vi "pharmaBot_v0.019.vi"() -> ()   [LabVIEW 2015] (continued)
  # "It saves the location when you push it -->"
  # "Set the Pipette Template"
  # "Click near the tip of the pipette in the @multiBot camera window then interface with the pop-up dialog to set the tip location and the pipette geometry.\n\nOnce complete, select the 'done' button below."
  # "Add Cells for Patching"
  # "Search around in the @multibot camera window and locate cells. Click on the center of desirable cells.\n\nOnce complete, select the 'done' button below."
  # "Calibration Complete"
  # "Stage"
  # "Manipulator"
  # "Select the Cell Index that you would like to add back into the \"unpatched cell indices\" array using the right and left arrow. To add the cell, click the Add Index to Unpatched Array Button. When finished, select done."
  # "CLEANING"
  # "EXPERIMENT SETTINGS"
  # "Voltage"
  # "NEURON DETECTION SETTINGS"
  # "Jumper"
  # "MACHINE VISION"
  # "DEBUGGING"
  # "MANIPULATOR 1"
  # "MANIPULATOR 2"
  # "CELL AUTOFOCUS"
  # "PIPETTE AUTOFOCUS"
  # "Position Set?"
  # "Jump Good?"
  # "HEK"
  # "SLICE"
  # "offset sets holding after membrane test..?"
  # "VERSION CONTROL\n\npharmaBot v0.009 - can't support dual patch but can control jumper\n\n9/9/17\nmultiBot v0.013 is compatible with multipatch_states_v0.013.\nColby's improved calibration routine is here. Adding pipette tracking verifier\n\n7/25/17\nmultiBot v0.011 is compatible with multipatch_states_v0.011: working on \ndual slice patching\n\n7-13-17\n- multiBot v0.010 is compatible with multipatch_states_v0.010. Latest stable version \nfor slice single patching and HEK cell dual patching\n\n7-6-17\nmultiBot v0.008 is compatible with multipatch_states_v0.008 AND v0.009\n- latest stable version - use for HEK and slices\n\n6/23/17\nmultiBot v0.007 is compatible with multipatch_states_v0.007\n- cell tracker working great\n- latest stable version for SINGLE-PATCH image tracking in slices\nmultiBot v0.006_reentrants is compatible with multipatch_states_wrapper_v0.001\nmultiBot v0.005 is compatible with multipatch_states_v0.005\nmultiBot v0.004 is compatible with multipatch_states_v0.004"
  # "TODO:\n\n- slow retractions for morphology\n- WC logic + recording software\n- simultaneous break-in\n- cell tracker for right pipette"
  # "@pharmaBot"
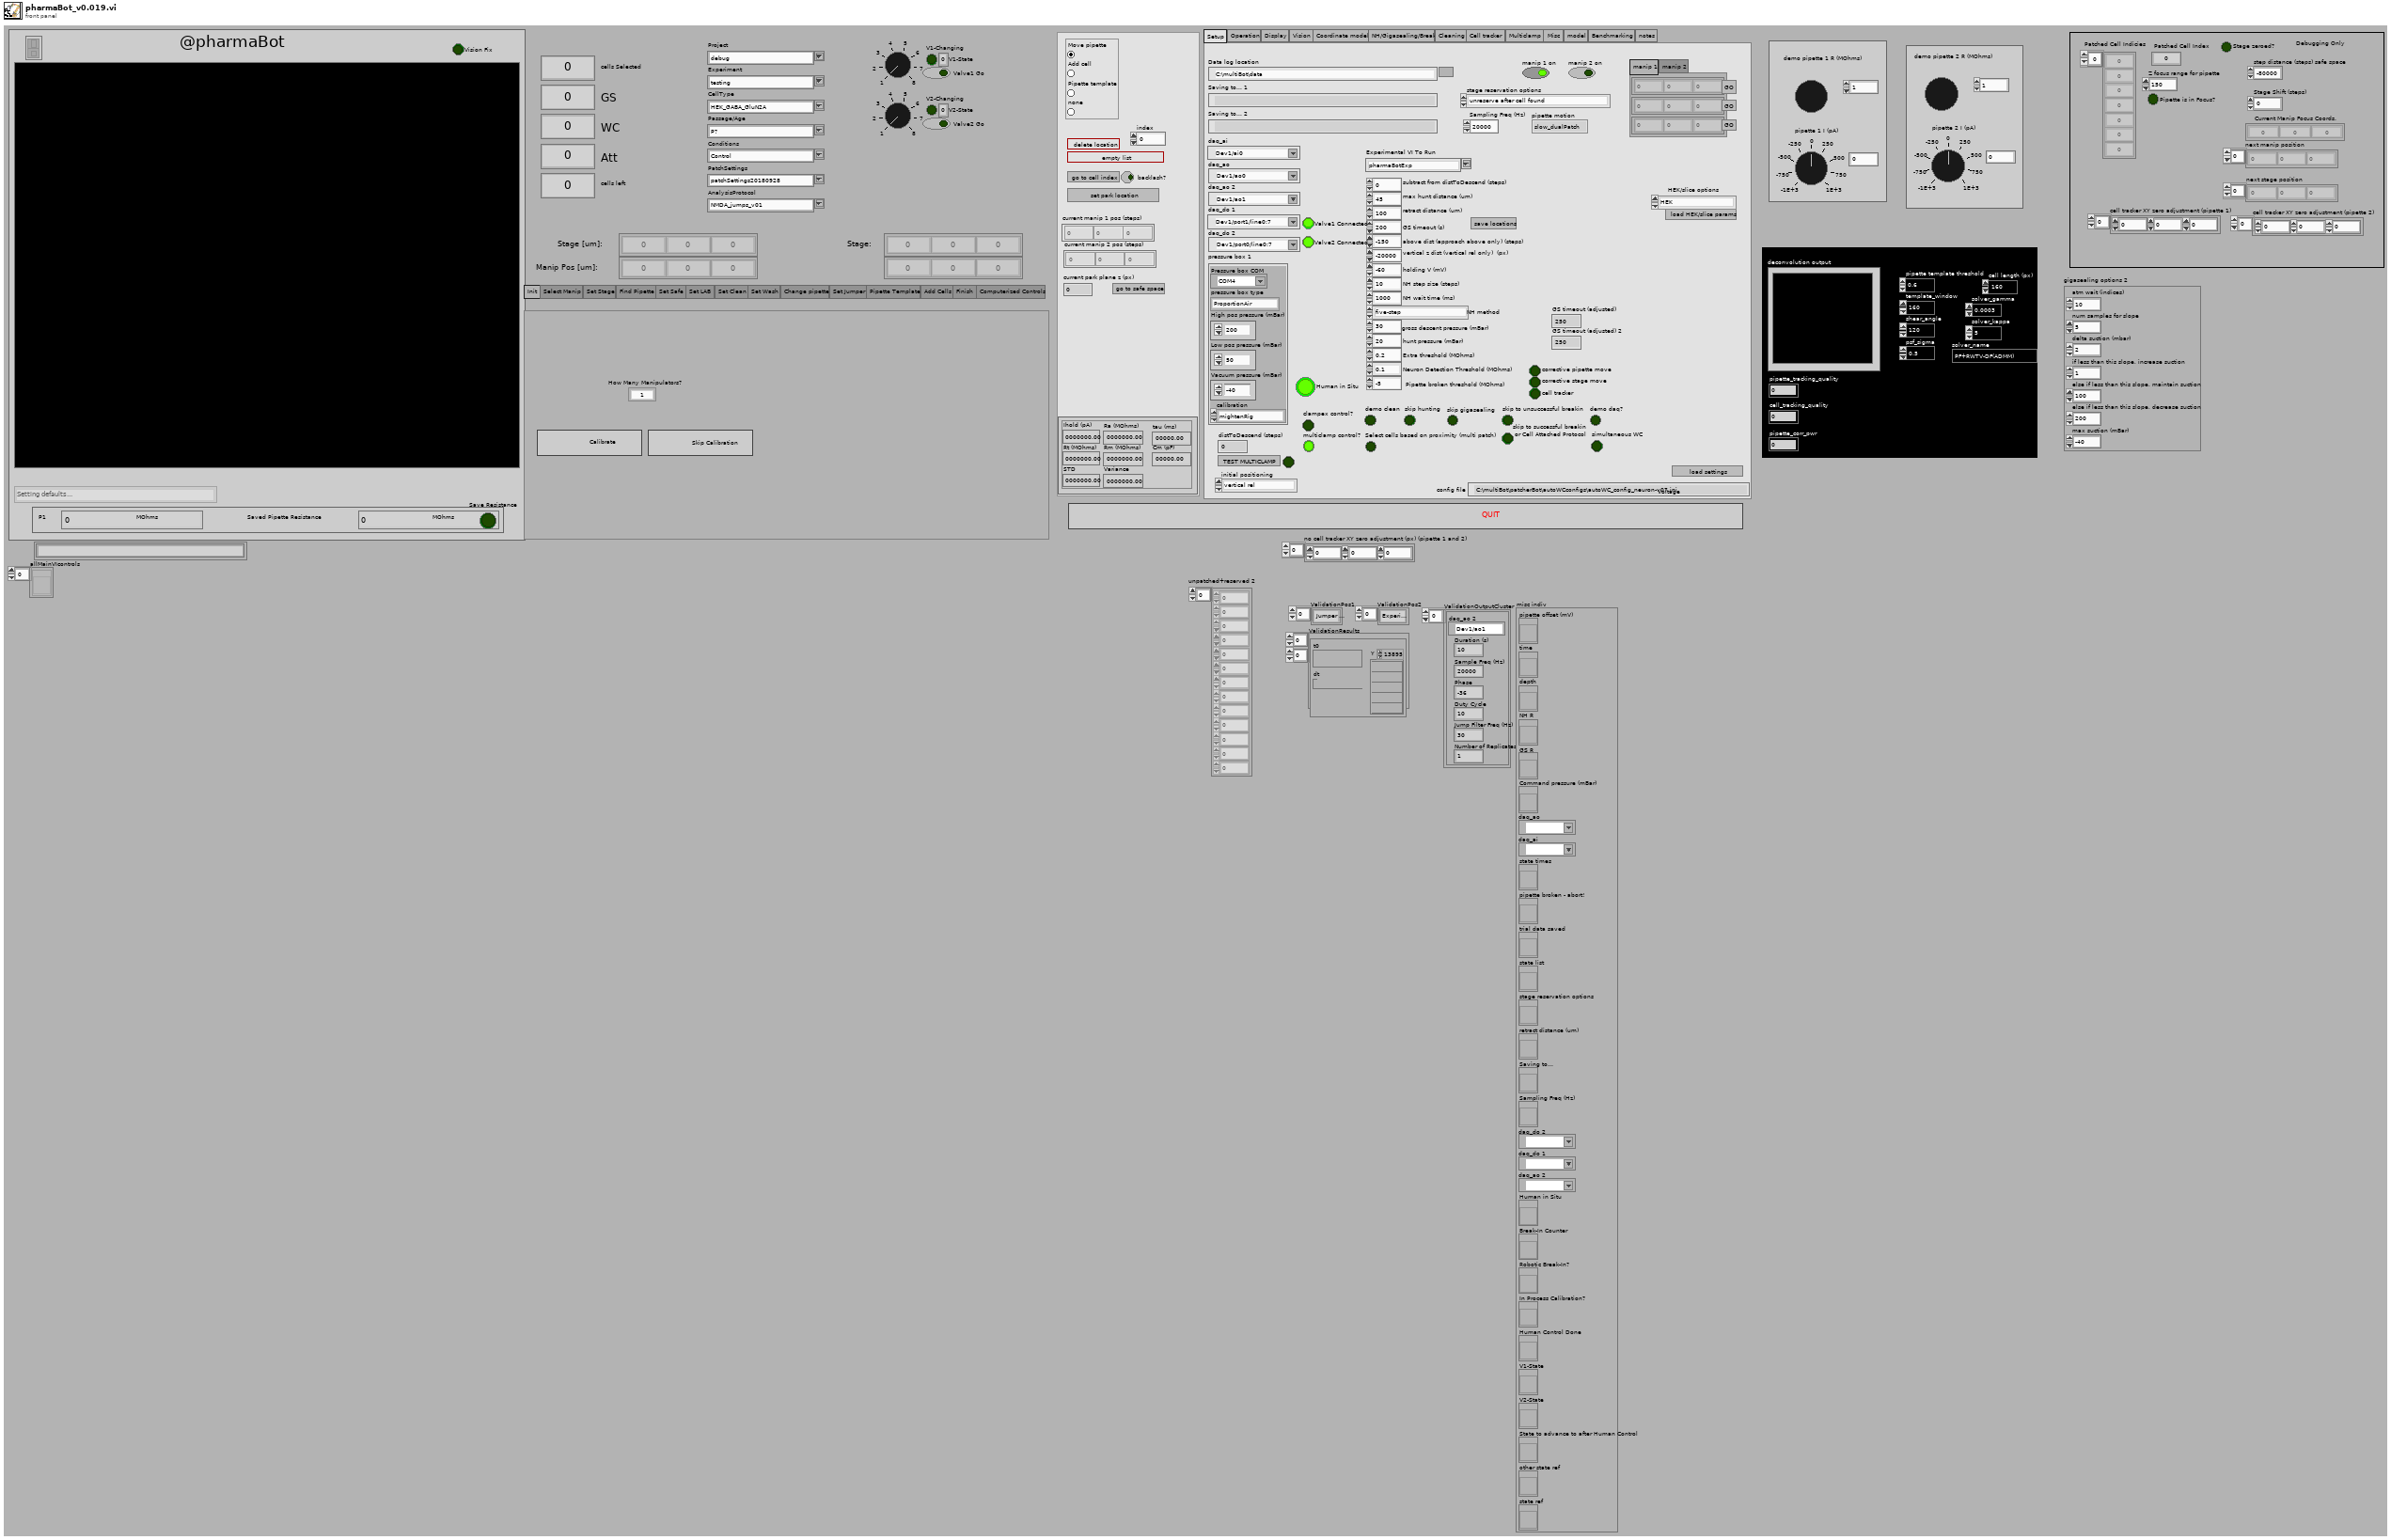
[diagram p1: front panel]
types:
  T1 = cluster{"pipette offset (mV)":refnum<vi>, "time":refnum<vi>, "depth":refnum<vi>, "NH R":refnum<vi>, "GS R":refnum<vi>, "Command pressure (mBar)":refnum<vi>, "daq_ao":tag, "daq_ai":tag, "state times":refnum<vi>, "pipette broken - abort!":refnum<vi>, "trial data saved":refnum<vi>, "state list":refnum<vi>, "stage reservation options":refnum<vi>, "retract distance (um)":refnum<vi>, "Saving to...":refnum<vi>, "Sampling Freq (Hz)":refnum<vi>, "daq_do 2":tag, "daq_do 1":tag, "daq_ao 2":tag, "Human in Situ":refnum<vi>, "Break-In Counter":refnum<vi>, "Robotic Break-In?":refnum<vi>, "In Process Calibration?":refnum<vi>, "Human Control Done":refnum<vi>, "V1-State":refnum<vi>, "V2-State":refnum<vi>, "State to advance to after Human Control":refnum<vi>, "other state ref":refnum<vi>, "state ref":refnum<vi>}
  T2 = cluster{"daq_ao 2":tag, "Duration (s)":dbl, "Sample Freq (Hz)":dbl, "Phase":dbl, "Duty Cycle":dbl, "Jump Filter Freq (Hz)":dbl, "Number of Replicates":i16}[]
  T3 = enum16{"Jumper Safe Position", "Experiment Safe Position", "Jumper Position A", "Jumper Position B", "Jumper Position C", "Jumper Position o-A", "Jumper Position A-o", "Jumper Position A-B", "Jumper Position B-A", "Jumper Position B-C", "Jumper Position C-B", "Jumper Position C-o", "Jumper Position o-C"}[]
  T4 = cluster{"atm wait (indices)":i32, "num samples for slope":i32, "delta suction (mbar)":dbl, "if less than this slope, increase suction":dbl, "else if less than this slope, maintain suction":dbl, "else if less than this slope, decrease suction ":dbl, "max suction (mBar)":dbl}
  T5 = typedef "cell_stats-v02.ctl" = cluster{"Ihold (pA)":dbl, "Rm (MOhms)":dbl, "Ra (MOhms)":dbl, "Cm (pF)":dbl, "tau (ms)":dbl, "Rt (MOhms)":dbl, "Variance":dbl, "STD":dbl}
  T6 = enum32{"Move pipette", "Add cell", "Pipette template", "none"}
  T7 = enum32{"Init", "Select Manip", "Set Stage", "Find Pipette", "Set Safe", "Set LAB", "Set Clean", "Set Wash", "Reset 0s", "Change pipette", "Set Jumper", "Pipette Template", "Add Cells", "Finish", "Computerized Controls", "Load Old Cells"}
  T8 = enum16{"manipulator 1", "manipulator 2", "manipulator 3", "manipulator 4"}
  T9 = enum16{"Jumper Safe Position", "Experiment Safe Position", "Jumper Position A", "Jumper Position B", "Jumper Position C", "Jumper Position o-A", "Jumper Position A-o", "Jumper Position A-B", "Jumper Position B-A", "Jumper Position B-C", "Jumper Position C-B", "Jumper Position C-o", "Jumper Position o-C"}
  T10 = typedef "IMAQ Image.ctl" = refnum<image>
  T11 = typedef "user_message_v6.ctl" = enum16{"Initializing...", "Setting defaults...", "Click OK to start patcherBot!", "Starting new attempt...", "Pipette repositioning...", "Initializing cell tracker...", "Gross approach...", "Human Positioning...", "In Process Calibration", "Detecting cell...", "Cell detected...", "Gigaseal Established...", "Breaking in...", "Successful breakin!", "Unsuccessful breakin!", "Whole-cell recording", "Saving autopatching parameters...", "Quitting VI", "Waiting for idle stage...", "Cleaning...", "Retracting pipette...", "DEBUG STATE", "Waiting to break in...", "Waiting for WC", "reclean", "Done with Current Set of Cells"}
  T12 = enum32{"Setup", "Operation", "Display", "Vision", "Coordinate model", "NH/Gigasealing/Break", "Cleaning", "Cell tracker", "Multiclamp", "Misc", "model", "Benchmarking", "notes"}
  T13 = typedef "Control 7b.ctl" = i32
  T14 = typedef "pressure_box_control.ctl" = cluster{"Pressure box COM":refnum<visa-resource-name>, "pressure box type":T15, "High pos pressure (mBar)":dbl, "Low pos pressure (mBar)":dbl, "Vacuum pressure (mBar)":dbl, "calibration":enum16{"PA_vacPump", "PA_venturi", "Neuromatics", "ilyaRig", "mightenRig"}}
  T15 = typedef "pressure_box_type.ctl" = enum16{"Neuromatics", "ProportionAir", "Demo box", "N-ProportionAir"}
  T16 = typedef "approach_type.ctl" = enum16{"right to cell", "vertical abs", "approach", "vertical rel", "approach above"}
  T17 = enum16{"unreserve after gross approach", "unreserve after cell found"}
  T18 = typedef "NH_method.ctl" = enum16{"five-step", "three-stepANDfixedCutOff", "three-step"}
  T19 = typedef "scope_motion.ctl" = enum16{"superSlow", "fast", "slow", "find slice speed", "slow_dualPatch"}
  T20 = typedef "notSureControl-v01.ctl" = bool
  T21 = cluster{"Starting Value":sgl, "Incremental Value":sgl, "Histogram":u32[]}
  T22 = typedef "cam_type-v02.ctl" = enum16{"HamamatsuORCA05G", "Qcam", "optiMOS"}
  T23 = cluster{"width x":dbl, "height y":dbl, "x offset":dbl, "y offset":dbl}
  T24 = enum32{"stage", "manip 1", "manip 2", "manip 3", "manip 4"}
  T25 = typedef "transform_properties_actuators.ctl" = cluster{"theta (deg)":dbl, "X sc factor (px/step)":dbl, "Y sc factor (px/step)":dbl, "zero loc (x,y,z)":dbl[], "flip y?":bool, "flip x?":bool, "gamma (deg)":dbl, "flip z?":bool, "Z sc factor (px/step)":dbl, "actuator":T26, "safe space (steps)":i32[]}
  T26 = typedef "actuator_cluster.ctl" = cluster{"Actuator COM":refnum<visa-resource-name>, "Actuator type":T27}
  T27 = typedef "actuator_type.ctl" = enum16{"Scientifica", "Sutter", "Demo", "Off"}
  T28 = typedef "ROI Descriptor" = cluster{"Global Rectangle":i32[], "Contours":cluster{"ID":enum32{"External", "Internal"}, "Type":u32, "Coordinates":i32[]}[]}
  T29 = typedef "memtest_def.ctl" = cluster{"Samples to Read":i32, "Rate (Hz)":dbl, "Amplitude (mV/pA)":dbl, "Offset (mV/pA)":dbl, "Frequency (Hz)":dbl, "duty cycle (%)":dbl, "phase":dbl}
  T30 = cluster{u32, string, i32, u32, u32, u32, "arg1":i32}
  T31 = enum16{"manipulator 1", "manipulator 2", "manipulator 3", "manipulator 4"}[]
  T32 = typedef "dual_patch_controls.ctl" = cluster{"sampling rate (Hz)":dbl, "total duration (s)":dbl, "stim amplitude (pA)":dbl, "time between stims (s)":dbl, "delta t (s)":dbl, "pulse width (s)":dbl, "# repetitions":dbl, "number of pulses":i32, "before stim (s)":dbl}
  T33 = cluster{"cells (image px locations)":dbl[], "cells (image px locations)":dbl[]}[]
  T34 = typedef "multipatch_individual_controls_v5.ctl" = cluster{"state UI indiv":cluster{"clampex control?":refnum<vi>, "demo clean":refnum<vi>, "skip hunting":refnum<vi>, "skip gigasealing":refnum<vi>, "multiclamp control?":refnum<vi>, "corrective pipette move":refnum<vi>, "corrective stage move":refnum<vi>, "cell tracker":refnum<vi>, "demo daq?":refnum<vi>, "skip to unsuccessful breakin":refnum<vi>, "skip to successful breakin":refnum<vi>, "successful breakin":refnum<vi>}, "positioning + hunting indiv":cluster{"NH step size (steps)":refnum<vi>, "hunt pressure (mBar)":refnum<vi>, "distToDescend (steps)":refnum<vi>, "approach above cell (steps)":refnum<vi>, "initial positioning":refnum<vi>, "d(above cell) (steps)":refnum<vi>, "neuron found":refnum<vi>, "NEURON HUNTING MONITOR":refnum<vi>, "Memtest inputs":refnum<vi>, "max hunt distance (um)":refnum<vi>, "Neuron Detection Threshold (MOhms)":refnum<vi>, "Pipette broken threshold (MOhms)":refnum<vi>, "gross descent pressure (mBar)":refnum<vi>, "Extra threshold (MOhms)":refnum<vi>, "current cell":refnum<vi>, "vertical z dist (vertical rel only)  (px)":refnum<vi>}, "gigaseal indiv":cluster{"GS timeout (s)":refnum<vi>, "GS timeout (adjusted)":refnum<vi>, "vhold applied?":refnum<vi>, "pipette resistance":refnum<vi>, "Iholding":refnum<vi>, "start GS time":refnum<vi>, "GIGASEALING MONITOR":refnum<vi>, "current Vholding (mV)":refnum<vi>, "GS extended":refnum<vi>, "holding V (mV)":refnum<vi>, "gigasealing options":refnum<vi>, "Cm":refnum<vi>, "Ra ":refnum<vi>}, "cleaning indiv":cluster{"pre-clean":refnum<vi>, "loc above baths":refnum<vi>, "wash bath loc":refnum<vi>, "cleaning bath loc":refnum<vi>, "cleaning status":refnum<vi>, "avg peak height":refnum<vi>, "clean bath detected":refnum<vi>, "wash bath detected":refnum<vi>}, "cell tracker indiv":cluster{"screen tip location (px)":refnum<vi>, "cell found":refnum<vi>, "tip found":refnum<vi>, "cell tracking box (px)":refnum<vi>}, "misc indiv":cluster{"pipette offset (mV)":refnum<vi>, "time":refnum<vi>, "depth":refnum<vi>, "NH R":refnum<vi>, "GS R":refnum<vi>, "Command pressure (mBar)":refnum<vi>, "daq_ao":tag, "daq_ai":tag, "state times":refnum<vi>, "pipette broken - abort!":refnum<vi>, "trial data saved":refnum<vi>, "state list":refnum<vi>, "stage reservation options":refnum<vi>, "retract distance (um)":refnum<vi>, "Saving to...":refnum<vi>, "Sampling Freq (Hz)":refnum<vi>, "daq_do 2":tag, "daq_do 1":tag, "daq_ao 2":tag, "Human in Situ":refnum<vi>, "Break-In Counter":refnum<vi>, "Robotic Break-In?":refnum<vi>, "In Process Calibration?":refnum<vi>, "Human Control Done":refnum<vi>, "V1-State":refnum<vi>, "V2-State":refnum<vi>, "State to advance to after Human Control":refnum<vi>, "other state ref":refnum<vi>, "state ref":refnum<vi>}, "breakin indiv":cluster{"breakin counter":refnum<vi>, "MAX Break In Pressure (mbar)":refnum<vi>}, "vision indiv":cluster{"manip position":refnum<vi>, "cell tracker XY zero adjustment (px)":refnum<vi>, "no cell tracker XY zero adjustment (px)":refnum<vi>}}
  T35 = cluster{"current stage pos (steps)":refnum<vi>, "current manip 1 pos (steps)":refnum<vi>, "current manip 2 pos (steps)":refnum<vi>, "current manip 3 pos (steps)":refnum<vi>, "current manip 4 pos (steps)":refnum<vi>}
  T36 = typedef "transform_cluster_actuator.ctl" = cluster{"s":refnum<vi>, "manip 1":refnum<vi>, "manip 2":refnum<vi>, "manip 3":refnum<vi>, "manip 4":refnum<vi>}
  T37 = typedef "multipatch_common_controls_v4.ctl" = cluster{"cell tracker common":cluster{"solver_beta":refnum<vi>, "solver_kappa":refnum<vi>, "shear_angle":refnum<vi>, "solver_gamma":refnum<vi>, "template_window":refnum<vi>, "debug_mode":refnum<vi>, "psf_sigma":refnum<vi>, "solver_name":refnum<vi>, "centroid_px":refnum<vi>, "pipette_px":refnum<vi>, "pipette_tracking_quality":refnum<vi>, "cell_tracking_quality":refnum<vi>, "pipette template threshold":refnum<vi>, "cell centroid array":refnum<vi>, "pipette centroid array":refnum<vi>, "cell length (px)":refnum<vi>}, "vision common":cluster{"init tracker success":refnum<vi>, "run tracker success":refnum<vi>, "tracking":refnum<vi>, "exit tracker success":refnum<vi>, "init error out":refnum<vi>, "current pipette locations (px)":refnum<vi>, "cell image size (px)":refnum<vi>, "pipette match score":refnum<vi>, "cell match score":refnum<vi>}, "misc common":cluster{"initialized":refnum<vi>, "Data log location":refnum<vi>, "Multiclamp Handle":refnum<vi>, "mclamp cluster":refnum<vi>, "User OK":refnum<vi>, "stage idle?":refnum<vi>, "stop":refnum<vi>, "pipette motion":refnum<vi>, "stop memtest":refnum<vi>, "dual patch cluster":refnum<vi>, "simultaneous WC":refnum<vi>, "Select cells based on proximity (multi patch)":refnum<vi>, "dual WC keep going":refnum<vi>, "HEK/slice options":refnum<vi>, "Terminate Experiment":refnum<vi>, "Validate":refnum<vi>}, "positioning+hunting common":cluster{"current cell locations (px)":refnum<vi>, "cells (image px)":refnum<vi>, "current park plane z (px)":refnum<vi>, "gross descent pressure (mBar)":refnum<vi>, "positions":refnum<vi>, "transforms":refnum<vi>, "pressure box":refnum<vi>, "current pipette locations (px)":refnum<vi>, "unpatched cell indices":refnum<vi>, "NH method":refnum<vi>, "NH wait time (ms)":refnum<vi>}, "ExperimentDescriptors":cluster{"Project":refnum<vi>, "AnalysisProtocol":refnum<vi>, "PatchSettings":refnum<vi>, "Passage/Age":refnum<vi>, "CellType":refnum<vi>, "Experiment":refnum<vi>, "Conditions":refnum<vi>, "ExperimentVIToRun":refnum<vi>}, "JumperPositions":cluster{"JumperPos o-C":refnum<vi>, "JumperPos C-o":refnum<vi>, "JumperPos C-B":refnum<vi>, "JumperPos B-C":refnum<vi>, "JumperPos B-A":refnum<vi>, "JumperPos A-B":refnum<vi>, "JumperPos A-o":refnum<vi>, "JumperPos o-A":refnum<vi>, "JumperPos C":refnum<vi>, "JumperPos B":refnum<vi>, "JumperPos A":refnum<vi>, "ExpSafePos":refnum<vi>, "jumperSafePos":refnum<vi>}, "PreviousValidationResults":cluster{"ValidationResults":refnum<vi>, "ValidationPos1":refnum<vi>, "ValidationPos2":refnum<vi>, "ValidationOutputCluster":refnum<vi>}}
  T38 = typedef "cam_info.ctl" = cluster{"camera type":T22, "cam handle":u32, "data handle":u32, "cam size":i32[]}
  T39 = cluster{"initialized":refnum<vi>, "Data log location":refnum<vi>, "Multiclamp Handle":refnum<vi>, "mclamp cluster":refnum<vi>, "User OK":refnum<vi>, "stage idle?":refnum<vi>, "stop":refnum<vi>, "pipette motion":refnum<vi>, "stop memtest":refnum<vi>, "dual patch cluster":refnum<vi>, "simultaneous WC":refnum<vi>, "Select cells based on proximity (multi patch)":refnum<vi>, "dual WC keep going":refnum<vi>, "HEK/slice options":refnum<vi>, "Terminate Experiment":refnum<vi>, "Validate":refnum<vi>}
  T40 = cluster{"init tracker success":refnum<vi>, "run tracker success":refnum<vi>, "tracking":refnum<vi>, "exit tracker success":refnum<vi>, "init error out":refnum<vi>, "current pipette locations (px)":refnum<vi>, "cell image size (px)":refnum<vi>, "pipette match score":refnum<vi>, "cell match score":refnum<vi>}
  T41 = cluster{"solver_beta":refnum<vi>, "solver_kappa":refnum<vi>, "shear_angle":refnum<vi>, "solver_gamma":refnum<vi>, "template_window":refnum<vi>, "debug_mode":refnum<vi>, "psf_sigma":refnum<vi>, "solver_name":refnum<vi>, "centroid_px":refnum<vi>, "pipette_px":refnum<vi>, "pipette_tracking_quality":refnum<vi>, "cell_tracking_quality":refnum<vi>, "pipette template threshold":refnum<vi>, "cell centroid array":refnum<vi>, "pipette centroid array":refnum<vi>, "cell length (px)":refnum<vi>}
  T42 = cluster{"Project":refnum<vi>, "AnalysisProtocol":refnum<vi>, "PatchSettings":refnum<vi>, "Passage/Age":refnum<vi>, "CellType":refnum<vi>, "Experiment":refnum<vi>, "Conditions":refnum<vi>, "ExperimentVIToRun":refnum<vi>}
  T43 = cluster{"current cell locations (px)":refnum<vi>, "cells (image px)":refnum<vi>, "current park plane z (px)":refnum<vi>, "gross descent pressure (mBar)":refnum<vi>, "positions":refnum<vi>, "transforms":refnum<vi>, "pressure box":refnum<vi>, "current pipette locations (px)":refnum<vi>, "unpatched cell indices":refnum<vi>, "NH method":refnum<vi>, "NH wait time (ms)":refnum<vi>}
  T44 = cluster{"GS timeout (s)":refnum<vi>, "GS timeout (adjusted)":refnum<vi>, "vhold applied?":refnum<vi>, "pipette resistance":refnum<vi>, "Iholding":refnum<vi>, "start GS time":refnum<vi>, "GIGASEALING MONITOR":refnum<vi>, "current Vholding (mV)":refnum<vi>, "GS extended":refnum<vi>, "holding V (mV)":refnum<vi>, "gigasealing options":refnum<vi>, "Cm 1":refnum<vi>, "Ra 1":refnum<vi>}
  T45 = cluster{"JumperPos o-C":refnum<vi>, "JumperPos C-o":refnum<vi>, "JumperPos C-B":refnum<vi>, "JumperPos B-C":refnum<vi>, "JumperPos B-A":refnum<vi>, "JumperPos A-B":refnum<vi>, "JumperPos A-o":refnum<vi>, "JumperPos o-A":refnum<vi>, "JumperPos C":refnum<vi>, "JumperPos B":refnum<vi>, "JumperPos A":refnum<vi>, "ExpSafePos":refnum<vi>, "jumperSafePos":refnum<vi>}
  T46 = cluster{"ValidationResults":refnum<vi>, "ValidationPos1":refnum<vi>, "ValidationPos2":refnum<vi>, "ValidationOutputCluster":refnum<vi>}
  T47 = typedef "Image Type" = u32
  T48 = cluster{"clampex control?":refnum<vi>, "demo clean":refnum<vi>, "skip hunting":refnum<vi>, "skip gigasealing":refnum<vi>, "multiclamp control?":refnum<vi>, "corrective pipette move":refnum<vi>, "corrective stage move":refnum<vi>, "cell tracker":refnum<vi>, "demo daq?":refnum<vi>, "skip to unsuccessful breakin":refnum<vi>, "skip to successful breakin":refnum<vi>, "successful breakin":refnum<vi>}
  T49 = cluster{"NH step size (steps)":refnum<vi>, "hunt pressure (mBar)":refnum<vi>, "distToDescend (steps)":refnum<vi>, "approach above cell (steps)":refnum<vi>, "initial positioning":refnum<vi>, "d(above cell) (steps)":refnum<vi>, "neuron found":refnum<vi>, "NEURON HUNTING MONITOR":refnum<vi>, "Memtest inputs":refnum<vi>, "max hunt distance (um)":refnum<vi>, "Neuron Detection Threshold (MOhms)":refnum<vi>, "Pipette broken threshold (MOhms)":refnum<vi>, "gross descent pressure (mBar)":refnum<vi>, "Extra threshold (MOhms)":refnum<vi>, "current cell":refnum<vi>, "vertical z dist (vertical rel only)  (px)":refnum<vi>}
  T50 = cluster{"pre-clean":refnum<vi>, "loc above baths":refnum<vi>, "wash bath loc":refnum<vi>, "cleaning bath loc":refnum<vi>, "cleaning status":refnum<vi>, "avg peak height":refnum<vi>, "clean bath detected":refnum<vi>, "wash bath detected":refnum<vi>}
  T51 = cluster{"screen tip location (px)":refnum<vi>, "cell found":refnum<vi>, "tip found":refnum<vi>, "cell tracking box (px)":refnum<vi>}
  T52 = cluster{"breakin counter":refnum<vi>, "MAX Break In Pressure (mbar)":refnum<vi>}
  T53 = typedef "arduino_pressure_setting.ctl" = enum16{"High Positive Pressure", "Low Positive Pressure", "Atmospheric Pressure", "Low Vacuum", "High Vacuum", "Break In", "Puff"}
  T54 = typedef "images_controls.ctl" = cluster{"slice image":T10, "pipette template":T10, "found pipette":T10, "pipette mask for cell tracker":T10, "cell images ref":refnum<vi>}
  T55 = cluster{"manip 1 position":refnum<vi>, "cell tracker XY zero adjustment (pipette 1)":refnum<vi>, "no cell tracker XY zero adjustment (px) (pipette 1 and 2)":refnum<vi>}
  T56 = enum8{"Enabled", "Disabled", "Disabled and Grayed Out"}
  T57 = enum32{"Init", "Select Manip", "Set Stage", "Find Pipette", "Set Safe", "Set LAB", "Set Clean", "Set Wash", "Reset 0s", "Set Jumper", "Pipette Template", "Add Cells", "Finish", "Load Old Cells"}
  T58 = enum32{"Linear", "Log", "Exp", "Square", "Square root", "Power X", "Power 1/X"}
  T59 = cluster{"Left":i32, "Top":i32, "Right":i32, "Bottom":i32}
  T60 = typedef "scientifica_commands.ctl" = enum16{"ANGLE", "INSET", "FIRST", "ZERO", "Pz", "P", "absz", "ACC", "TOP", "STOP", "rel", "relz", "abs", "IN", "vj", "APROACH", "OBJS", "OBJU", "OUT", "OBJ", "OBJL", "SET", "OBJD", "STEP", "SETSTEP", "S", "UUX", "UUY", "UUZ"}
  T61 = enum16{"open", "replace", "create", "open or create", "replace or create", "replace or create with confirmation"}
  T62 = typedef "RWC_Actions.ctl" = enum16{"Read", "Write", "Read and Create"}
  T63 = cluster{"daq_ao 2":tag, "Duration (s)":dbl, "Sample Freq (Hz)":dbl, "Phase":dbl, "Duty Cycle":dbl, "Jump Filter Freq (Hz)":dbl, "Number of Replicates":i16}
diagram:
  w295 = T40 {"init tracker success"=refnum, "run tracker success"=refnum, "tracking"=refnum, "exit tracker success"=refnum, "init error out"=refnum, "current pipette locations (px)"=refnum, "cell image size (px)"=refnum, "pipette match score"=refnum, "cell match score"=refnum}  # vision common
  w296 = T41 {"solver_beta"=refnum, "solver_kappa"=refnum, "shear_angle"=refnum, "solver_gamma"=refnum, "template_window"=refnum, "debug_mode"=refnum, "psf_sigma"=refnum, "solver_name"=refnum, "centroid_px"=refnum, "pipette_px"=refnum, "pipette_tracking_quality"=refnum, "cell_tracking_quality"=refnum, "pipette template threshold"=refnum, "cell centroid array"=refnum, "pipette centroid array"=refnum, "cell length (px)"=refnum}  # cell tracker common
  w297 = T42 {"Project"=refnum, "AnalysisProtocol"=refnum, "PatchSettings"=refnum, "Passage/Age"=refnum, "CellType"=refnum, "Experiment"=refnum, "Conditions"=refnum, "ExperimentVIToRun"=refnum}  # ExperimentDescriptors
  w298 = T43 {"current cell locations (px)"=refnum, "cells (image px)"=refnum, "current park plane z (px)"=refnum, "gross descent pressure (mBar)"=refnum, "positions"=refnum, "transforms"=refnum, "pressure box"=refnum, "current pipette locations (px)"=refnum, "unpatched cell indices"=refnum, "NH method"=refnum, "NH wait time (ms)"=refnum}  # positioning+hunting common
  w299 = T44 {"GS timeout (s)"=refnum, "GS timeout (adjusted)"=refnum, "vhold applied?"=refnum, "pipette resistance"=refnum, "Iholding"=refnum, "start GS time"=refnum, "GIGASEALING MONITOR"=refnum, "current Vholding (mV)"=refnum, "GS extended"=refnum, "holding V (mV)"=refnum, "gigasealing options"=refnum, "Cm 1"=refnum, "Ra 1"=refnum}  # gigaseal indiv
  w300 = T45 {"JumperPos o-C"=refnum, "JumperPos C-o"=refnum, "JumperPos C-B"=refnum, "JumperPos B-C"=refnum, "JumperPos B-A"=refnum, "JumperPos A-B"=refnum, "JumperPos A-o"=refnum, "JumperPos o-A"=refnum, "JumperPos C"=refnum, "JumperPos B"=refnum, "JumperPos A"=refnum, "ExpSafePos"=refnum, "jumperSafePos"=refnum}  # jumperPositions
  w365 = T47 0 items=["Grayscale (U8)", "Grayscale (I16)", "Grayscale (SGL)", "Complex (CSG)", "RGB (U32)", "HSL (U32)", "RGB (U64)", "Grayscale (U16)"] ("Image Type")
  w426 = T50 {"pre-clean"=refnum, "loc above baths"=refnum, "wash bath loc"=refnum, "cleaning bath loc"=refnum, "cleaning status"=refnum, "avg peak height"=refnum, "clean bath detected"=refnum, "wash bath detected"=refnum}  # cleaning indiv
  w453 = dbl[][] [] ("appended array")
  w457 = 0 items=["All", "Low Discrepancy Sampling", "Grayscale Value Pyramid", "Gradients Pyramid"] ("Algorithm")
  w440 = T8."manipulator 2" ("which manipulator")
  w444 = T8."manipulator 1" ("which manipulator")
  w517 = T51 {"screen tip location (px)"=refnum, "cell found"=refnum, "tip found"=refnum, "cell tracking box (px)"=refnum}  # cell tracker indiv
  w478 = 0 ("current cell")
  w262 = FALSE ("extend GS")
  w263 = dbl[] [] ("state times")
  w521 = FALSE ("initialized?")
  w523 = T52 {"breakin counter"=refnum, "MAX Break In Pressure (mbar)"=refnum}  # breakin indiv
  w578 = T34 {"state UI indiv"={"clampex control?"=refnum, "demo clean"=refnum, "skip hunting"=refnum, "skip gigasealing"=refnum, "multiclamp control?"=refnum, "corrective pipette move"=refnum, "corrective stage move"=refnum, "cell tracker"=refnum, "demo daq?"=refnum, "skip to unsuccessful breakin"=refnum, "skip to successful breakin"=refnum, "successful breakin"=refnum}, "positioning + hunting indiv"={"NH step size (steps)"=refnum, "hunt pressure (mBar)"=refnum, "distToDescend (steps)"=refnum, "approach above cell (steps)"=refnum, "initial positioning"=refnum, "d(above cell) (steps)"=refnum, "neuron found"=refnum, "NEURON HUNTING MONITOR"=refnum, "Memtest inputs"=refnum, "max hunt distance (um)"=refnum, "Neuron Detection Threshold (MOhms)"=refnum, "Pipette broken threshold (MOhms)"=refnum, "gross descent pressure (mBar)"=refnum, "Extra threshold (MOhms)"=refnum, "current cell"=refnum, "vertical z dist (vertical rel only)  (px)"=refnum}, "gigaseal indiv"={"GS timeout (s)"=refnum, "GS timeout (adjusted)"=refnum, "vhold applied?"=refnum, "pipette resistance"=refnum, "Iholding"=refnum, "start GS time"=refnum, "GIGASEALING MONITOR"=refnum, "current Vholding (mV)"=refnum, "GS extended"=refnum, "holding V (mV)"=refnum, "gigasealing options"=refnum, "Cm"=refnum, "Ra "=refnum}, "cleaning indiv"={"pre-clean"=refnum, "loc above baths"=refnum, "wash bath loc"=refnum, "cleaning bath loc"=refnum, "cleaning status"=refnum, "avg peak height"=refnum, "clean bath detected"=refnum, "wash bath detected"=refnum}, "cell tracker indiv"={"screen tip location (px)"=refnum, "cell found"=refnum, "tip found"=refnum, "cell tracking box (px)"=refnum}, "misc indiv"={"pipette offset (mV)"=refnum, "time"=refnum, "depth"=refnum, "NH R"=refnum, "GS R"=refnum, "Command pressure (mBar)"=refnum, "daq_ao"="", "daq_ai"="", "state times"=refnum, "pipette broken - abort!"=refnum, "trial data saved"=refnum, "state list"=refnum, "stage reservation options"=refnum, "retract distance (um)"=refnum, "Saving to..."=refnum, "Sampling Freq (Hz)"=refnum, "daq_do 2"="", "daq_do 1"="", "daq_ao 2"="", "Human in Situ"=refnum, "Break-In Counter"=refnum, "Robotic Break-In?"=refnum, "In Process Calibration?"=refnum, "Human Control Done"=refnum, "V1-State"=refnum, "V2-State"=refnum, "State to advance to after Human Control"=refnum, "other state ref"=refnum, "state ref"=refnum}, "breakin indiv"={"breakin counter"=refnum, "MAX Break In Pressure (mbar)"=refnum}, "vision indiv"={"manip position"=refnum, "cell tracker XY zero adjustment (px)"=refnum, "no cell tracker XY zero adjustment (px)"=refnum}}  # individual controls
  w583 = T37 {"cell tracker common"={"solver_beta"=refnum, "solver_kappa"=refnum, "shear_angle"=refnum, "solver_gamma"=refnum, "template_window"=refnum, "debug_mode"=refnum, "psf_sigma"=refnum, "solver_name"=refnum, "centroid_px"=refnum, "pipette_px"=refnum, "pipette_tracking_quality"=refnum, "cell_tracking_quality"=refnum, "pipette template threshold"=refnum, "cell centroid array"=refnum, "pipette centroid array"=refnum, "cell length (px)"=refnum}, "vision common"={"init tracker success"=refnum, "run tracker success"=refnum, "tracking"=refnum, "exit tracker success"=refnum, "init error out"=refnum, "current pipette locations (px)"=refnum, "cell image size (px)"=refnum, "pipette match score"=refnum, "cell match score"=refnum}, "misc common"={"initialized"=refnum, "Data log location"=refnum, "Multiclamp Handle"=refnum, "mclamp cluster"=refnum, "User OK"=refnum, "stage idle?"=refnum, "stop"=refnum, "pipette motion"=refnum, "stop memtest"=refnum, "dual patch cluster"=refnum, "simultaneous WC"=refnum, "Select cells based on proximity (multi patch)"=refnum, "dual WC keep going"=refnum, "HEK/slice options"=refnum, "Terminate Experiment"=refnum, "Validate"=refnum}, "positioning+hunting common"={"current cell locations (px)"=refnum, "cells (image px)"=refnum, "current park plane z (px)"=refnum, "gross descent pressure (mBar)"=refnum, "positions"=refnum, "transforms"=refnum, "pressure box"=refnum, "current pipette locations (px)"=refnum, "unpatched cell indices"=refnum, "NH method"=refnum, "NH wait time (ms)"=refnum}, "ExperimentDescriptors"={"Project"=refnum, "AnalysisProtocol"=refnum, "PatchSettings"=refnum, "Passage/Age"=refnum, "CellType"=refnum, "Experiment"=refnum, "Conditions"=refnum, "ExperimentVIToRun"=refnum}, "JumperPositions"={"JumperPos o-C"=refnum, "JumperPos C-o"=refnum, "JumperPos C-B"=refnum, "JumperPos B-C"=refnum, "JumperPos B-A"=refnum, "JumperPos A-B"=refnum, "JumperPos A-o"=refnum, "JumperPos o-A"=refnum, "JumperPos C"=refnum, "JumperPos B"=refnum, "JumperPos A"=refnum, "ExpSafePos"=refnum, "jumperSafePos"=refnum}, "PreviousValidationResults"={"ValidationResults"=refnum, "ValidationPos1"=refnum, "ValidationPos2"=refnum, "ValidationOutputCluster"=refnum}}  # common controls
  w625 = FALSE ("tracking")
  w631 = 0 items=["All", "Low Discrepancy Sampling", "Grayscale Value Pyramid", "Gradients Pyramid"] ("Algorithm")
  w536 = dbl[] [688.0, 512.0, 0.0] ("zero loc (x,y,z)")
  w648 = T47 7 items=["Grayscale (U8)", "Grayscale (I16)", "Grayscale (SGL)", "Complex (CSG)", "RGB (U32)", "HSL (U32)", "RGB (U64)", "Grayscale (U16)"] ("Image Type")
  w652 = T47 7 items=["Grayscale (U8)", "Grayscale (I16)", "Grayscale (SGL)", "Complex (CSG)", "RGB (U32)", "HSL (U32)", "RGB (U64)", "Grayscale (U16)"] ("Image Type")
  w332 = T47 7 items=["Grayscale (U8)", "Grayscale (I16)", "Grayscale (SGL)", "Complex (CSG)", "RGB (U32)", "HSL (U32)", "RGB (U64)", "Grayscale (U16)"] ("Image Type")
  w433 = T47 7 items=["Grayscale (U8)", "Grayscale (I16)", "Grayscale (SGL)", "Complex (CSG)", "RGB (U32)", "HSL (U32)", "RGB (U64)", "Grayscale (U16)"] ("Image Type")
  w474 = arduino_pressure_setting."Low Positive Pressure" ("pressure setting")
  w696 = path "C:/multiBot/ComputerSpecificSettingsAndDefaults/config/default_locations_multiBot.loc" ("file path (use dialog)")
  w518 = user_message_v6."Initializing..." ("Message to user")
  # "individual 1"
  # "individual  1"
  # "common"
  # "JUMPER POSITIONS"
  # "Jumper Positions"
  # "CAM Info"
  # "FOR QUAD PATCH\nadd manipulator 3 and 4"
  # "replicate this 2x more times for QUAD PATCH"
  # "get stage and manipulator positions\nFOR QUAD PATCH\nadd two more instances"
  # "FOR QUAD PATCHING\nthis needs to output 4 pipette ressitances and currents and peak heights"
  # "current positions"
  # "3D MODEL\nupdates cell locations"
  # "USER INTERFACE"
  # "DAQ loop"
  # "CELL TRACKER"
  # "CAMERA"
  # "COMMON"
  # "INDIVIDUAL 2"
  # "IMAGES 2"
  # "misc\nINDIVIDUAL\n2"
  # "IMAGES 1"
  # "INDIVIDUAL 1"
  # "COMMON"
  # "TRANSFORMS"
  # "POSITIONS"
  # "MANIP 2 INDIVIDUAL CONTROLS"
  # "USER CONTROLS"
  # "AMPLIFIER"
  # "MISC"
  # "BREAKIN"
  # "HUNTING"
  # "POSITIONING"
  # "CLEANING"
  # "VISION"
  # "CELL TRACKER"
  # "vision\nINDIVIDUAL"
  # "breakin\nINDIVIDUAL"
  # "DUPLICATE\nTHIS \nFOR\nPIPETTE\n2!!"
  # "positioning/hunting\nINDIVIDUAL"
  # "cell tracker\nINDIVIDUAL"
  # "positioning/hunting\nCOMMON"
  # "cleaning\nINDIVIDUAL"
  # "misc\nINDIVIDUAL"
  # "misc\nCOMMON"
  # "gigaseal\nINDIVIDUAL"
  # "vision\nCOMMON"
  # "cell tracker controls\nCOMMON"
  # "state UI controls\nINDIVIDUAL"
  # "reset zero position"
  # "MATLAB RUN LOOP"
  # "create image buffer"
  # "pressure"
  # "slice view"
  # "delete image buffer"
  # "create image buffer"
  # "delete image buffer"
  # "INITIALIZATION"
  # "make sure the quit button is reset"
  # "Route all error signals from initialization here"
  # "multiclamp initialization\nFOR QUAD PATCH\nhow to add another Multiclamp"
  n1 = control-ref of="Power Spectrum inputs"() -> (w6:refnum<vi>)
  n2 = control-ref of="demo daq?"() -> (w238:refnum<vi>)
  n3 = control-ref of="holding V (mV)"() -> (w218:refnum<vi>)
  n4 = control-ref of="Experimental VI To Run"() -> (w211:refnum<vi>)
  n5 = control-ref of="Conditions"() -> (w210:refnum<vi>)
  n6 = control-ref of="AnalysisProtocol"() -> (w209:refnum<vi>)
  n7 = control-ref of="PatchSettings"() -> (w208:refnum<vi>)
  n8 = control-ref of="Passage/Age"() -> (w207:refnum<vi>)
  n9 = control-ref of="CellType"() -> (w206:refnum<vi>)
  n10 = control-ref of="Experiment"() -> (w205:refnum<vi>)
  n11 = control-ref of="Project"() -> (w204:refnum<vi>)
  n12 = control-ref of="pipette motion"() -> (w237:refnum<vi>)
  n13 = control-ref of="daq_ao 2"() -> (w221:refnum<vi>)
  n14 = control-ref of="daq_ao"() -> (w220:refnum<vi>)
  n15 = control-ref of="daq_ai"() -> (w219:refnum<vi>)
  n16 = control-ref of="individual controls manip 2"() -> (w217:refnum<vi>)
  n17 = control-ref of="individual controls manip 1"() -> (w216:refnum<vi>)
  n18 = control-ref of="common controls"() -> (w215:refnum<vi>)
  n19 = control-ref of="stage->cam"() -> (w214:refnum<vi>)
  n20 = control-ref of="manip2->cam"() -> (w213:refnum<vi>)
  n21 = control-ref of="manip1->cam"() -> (w212:refnum<vi>)
  n22 = control-ref of="gigasealing options 2"() -> (w203:refnum<vi>)
  n23 = control-ref of="manip3->cam"() -> (w202:refnum<vi>)
  n24 = control-ref of="current manip 1 pos (steps)"() -> (w201:refnum<vi>)
  n25 = control-ref of="current manip 2 pos (steps)"() -> (w200:refnum<vi>)
  n26 = control-ref of="manip4->cam"() -> (w199:refnum<vi>)
  n27 = control-ref of="current manip 3 pos (steps)"() -> (w198:refnum<vi>)
  n28 = control-ref of="current manip 4 pos (steps)"() -> (w197:refnum<vi>)
  n29 = control-ref of="initial positioning"() -> (w196:refnum<vi>)
  n30 = control-ref of="distToDescend (steps)"() -> (w195:refnum<vi>)
  n31 = control-ref of="cell length (px)"() -> (w194:refnum<vi>)
  n32 = control-ref of="tracking"() -> (w193:refnum<vi>)
  n33 = control-ref of="cell tracking box (px)"() -> (w192:refnum<vi>)
  n34 = control-ref of="cell tracker"() -> (w191:refnum<vi>)
  n35 = control-ref of="pipette offset (mV)"() -> (w185:refnum<vi>)
  n36 = control-ref of="retract distance (um)"() -> (w184:refnum<vi>)
  n37 = control-ref of="above dist (approach above only) (steps)"() -> (w183:refnum<vi>)
  n38 = control-ref of="gross descent pressure (mBar)"() -> (w182:refnum<vi>)
  n39 = control-ref of="vertical z dist (vertical rel only)  (px)"() -> (w181:refnum<vi>)
  n40 = control-ref of="unpatched cell indices"() -> (w180:refnum<vi>)
  n41 = control-ref of="cam size"() -> (w239:refnum<vi>)